vi "UHR-Fleezers Control (host) - 12.7e.vi"() -> ()   [LabVIEW 2012] (continued)
        n405 = And(x="Trap 1 ON", y=w546) -> (x .and. y?=w544:bool)
        n406 = Multiply(x=w558, y=w569) -> (x*y=w566:dbl)
        n407 = Multiply(x=w568, y=w557) -> (x*y=w564:dbl)
        n408 = Multiply(x=w567, y=w556) -> (x*y=w565:dbl)
        n409 = Multiply(x=w570, y=w555) -> (x*y=w573:dbl)
        n410 = Multiply(x=w571, y=w554) -> (x*y=w574:dbl)
        n411 = Multiply(x=w572, y=w553) -> (x*y=w575:dbl)
        n412 = call "set RF board amplitude - interlace.vi"("Board 2 Amplitude Limits"=w539, "Board 1 Amplitude Limits"=w540, "FPGA VI Reference In"=w538, "Board 2 Amplitude 3 (%)"=w575, "Board 1 Amplitude 3 (%)"=w565, "Board 2 Amplitude 2 (%)"=w574, "Board 2 Amplitude 1 (%)"=w573, "Board 1 Amplitude 2 (%)"=w564, "Board 1 Amplitude 1 (%)"=w566) -> ("error out"=w548:errorcluster, "FPGA VI Reference Out"=w549:T20)  [unwired: 1 in]
        n413 = xnode "Read/Write Control"("FPGA VI Reference In"=w549, "error in"=w548, "FB On/Off Set 1"=w544, "FB On/Off Set 2"=w541) -> ("error out"=w547:errorcluster)  [unwired: 1 out]
      }
      event "Load parameters": Value Change {
        n414 = event-data() -> ()  [unwired: 7 out]
        n415 = property on="Saved AOD Raster Scan Parameter Sets" class="Arr (strict)"() -> ("Index Values"=w586:u32[])  [unwired: 2 in, 2 out]
        n416 = Index Array(array=w586, index=0) -> (element=w583:u32)
        n417 = local write "Load parameters"(FALSE ("Load parameters")) -> ()
        n418 = Index Array(array="Saved AOD Raster Scan Parameter Sets", index=w583) -> (element=w582:T28)
        n419 = Unbundle By Name(w582) -> ("Scan Range AOD (nm) 2"=w581:dbl, "Step Size AOD (nm) 2"=w580:dbl, "Scan Speed AOD (nm/s) 2"=w579:dbl, "Number of scans (AOD) 2"=w578:u16)
        n420 = flat-sequence {
          tunnel: w581 -> [w589]
          tunnel: w580 -> [w588]
          tunnel: w579 -> [w587]
          tunnel: w578 -> [w590]
          frame #0 {
            n421 = local write "Scan Speed (nm/s)"(w587) -> ()
            n422 = local write "Scan Range (nm)"(w589) -> ()
            n423 = local write "Step Size (nm)"(w588) -> ()
          }
          frame #1 {
            n424 = property on="Number of F/B Scans (AOD)" class="DigNum (strict)"("Val(Sgnl)"=w590) -> ()  [unwired: 2 in, 2 out]
          }
        }
      }
      event "Trap 1 (ON/OFF)", "Trap 2 (ON/OFF)": Value Change {
        n425 = event-data() -> ()  [unwired: 7 out]
        n426 = property on="Trap 2 ON" class="Bool (strict)"("Val(Sgnl)"="Trap 2 (ON/OFF)") -> ()  [unwired: 2 in, 2 out]
        n427 = property on="Trap 1 ON" class="Bool (strict)"("Val(Sgnl)"="Trap 1 (ON/OFF)") -> ()  [unwired: 2 in, 2 out]
      }
      event "DIO count 1 (ticks)", "DIO count 2 (ticks)", "DIO count 3 (ticks)", "Interlace", "Number Interlace Sets", "Not-Interlacing Set", "BD 1 Delay (ticks)", "BD 2 Delay (Ticks)", "Next trap write delay (ticks)", "XY phase ext loop method", "Amp switch delay 2", "BD 2 Delay (Ticks) 2", "BD 1 Delay (ticks) 2": Value Change {
        n428 = event-data() -> ()  [unwired: 7 out]
        n429 = local read "DIO count 3 (ticks)"() -> (w611:u16)
        n430 = local read "DIO count 1 (ticks)"() -> (w613:u16)
        n431 = local read "DIO count 2 (ticks)"() -> (w612:u16)
        n432 = To Unsigned Byte Integer(number="Not-Interlacing Set") -> (unsigned 8bit integer=w602:u8)
        n433 = Add(x=w602, y=u8 1) -> (x+y=w606:u8)
        n434 = xnode "Read/Write Control"("FPGA VI Reference In"=w593, "DIO count 1 (ticks)"=w613, "DIO count 2 (ticks)"=w612, "DIO count 3 (ticks)"=w611, "Interlace ON/OFF"="Interlace", "Number Interlace Cycles"="Number Interlace Sets", "Interlace Off Parameters"=w606, "BD 1 Delay (ticks)"="BD 1 Delay (ticks)", "BD 2 Delay (Ticks)"="BD 2 Delay (Ticks)", "Next trap write delay (ticks)"="Next trap write delay (ticks)", "XY phase ext loop method"="XY phase ext loop method", "Amp switch delay 2"="Amp switch delay 2", "BD 2 Delay (Ticks) 2"="BD 2 Delay (Ticks) 2", "BD 1 Delay (ticks) 2"="BD 1 Delay (ticks) 2") -> ("error out"=w615:errorcluster)  [unwired: 1 in, 1 out]
        n435 = Build Array(w613, w612, w611) -> (w604:u16[])
        n436 = Split 1D Array(array=w604, index="Number Interlace Sets") -> (first subarray=w614:u16[])  [unwired: 1 out]
        n437 = Index Array(array=w604, index=w602) -> (element=w603:u16)
        n438 = Add Array Elements(numeric array=w614) -> (sum=w608:u16)
        n439 = Select(t=w608, s="Interlace", f=w603) -> (s? t:f=→"Total Counts (ticks)":u16)
      }
      event "Reset Feedback": Value Change {
        n440 = event-data() -> ()  [unwired: 7 out]
        n441 = Unbundle By Name("Reset Feedback") -> ("Set 1"=w619:bool, "Set 2"=w618:bool)
        n442 = xnode "Read/Write Control"("FPGA VI Reference In"=w616, "FB Reset Set 1"=w619, "FB Reset Set 2"=w618) -> ("error out"=w617:errorcluster)  [unwired: 1 in, 1 out]
      }
      event "Trap Intensity PID Gains": Value Change {
        n443 = event-data() -> ()  [unwired: 7 out]
        n444 = Unbundle By Name("Trap Intensity PID Gains") -> ("proportional gain (Kc)"=w624:i16, "integral gain (Kc*Ts/Ti)"=w623:i16, "derivative gain (Kc*Td/Ts)"=w622:i16)
        n445 = xnode "Read/Write Control"("FPGA VI Reference In"=w621, "P1"=w624, "I1"=w623, "D1"=w622) -> ("error out"=w626:errorcluster)  [unwired: 1 in, 1 out]
      }
      event "AI2 to Setpoint", "Setpoints (V)": Value Change {
        n446 = event-data() -> ()  [unwired: 7 out]
        n447 = xnode "Read/Write Control"("FPGA VI Reference In"=w627) -> ("FPGA VI Reference Out"=w630:T20, "error out"=w629:errorcluster, "AI2 Y Sum Set 1"=w637:i16, "AI2 Y Sum Set 2"=w636:i16)  [unwired: 1 in]
        n448 = Cluster To Array(cluster="AI2 to Setpoint") -> (array=w640:bool[])
        n449 = local read "AI2 (V)"() -> (w638:cluster{"Set 1":dbl, "Set 2":dbl})
        n450 = Or Array Elements(Boolean array=w640) -> (logical OR=w641:bool)
        n451 = Bundle By Name(cluster=w638, "Set 1"=w637, "Set 2"=w636) -> (w635:cluster{"Set 1":dbl, "Set 2":dbl})
        n452 = Divide(x=w635, y=3276.7) -> (x/y=w634:cluster{"Set 1":dbl, "Set 2":dbl})
        "AI2 (V)" <- w634
        n453 = case shown="True" w641 {
          tunnel: [w644 w661] -> w633
          tunnel: "AI2 to Setpoint" -> [_ w657]
          tunnel: "Setpoints (V)" -> [w645 w660]
          tunnel: w634 -> [_ w654]
          frame False {
            n454 = Multiply(x=3276.7, y=w645) -> (x*y=w646:cluster{"Set 1":dbl, "Set 2":dbl})
            n455 = To Word Integer(number=w646) -> (16bit integer=w644:cluster{"Set 1":i16, "Set 2":i16})
          }
          frame True {
            n456 = Unbundle By Name(w654) -> ("Set 1"=w653:dbl, "Set 2"=w652:dbl)
            n457 = Unbundle By Name(w660) -> ("Set 1"=w659:dbl, "Set 2"=w658:dbl)
            n458 = Unbundle By Name(w657) -> ("Set 1"=w656:bool, "Set 2"=w655:bool)
            n459 = Select(t=w653, s=w656, f=w659) -> (s? t:f=w651:dbl)
            n460 = Select(t=w652, s=w655, f=w658) -> (s? t:f=w650:dbl)
            n461 = Bundle By Name(cluster=w660, "Set 1"=w651, "Set 2"=w650) -> (w648:cluster{"Set 1":dbl, "Set 2":dbl})
            n462 = local write "Setpoints (V)"(w648) -> ()
            n463 = Multiply(x=3276.7, y=w648) -> (x*y=w649:cluster{"Set 1":dbl, "Set 2":dbl})
            n464 = To Word Integer(number=w649) -> (16bit integer=w661:cluster{"Set 1":i16, "Set 2":i16})
          }
        }
        n465 = Unbundle By Name(w633) -> ("Set 1"=w632:i16, "Set 2"=w631:i16)
        n466 = xnode "Read/Write Control"("FPGA VI Reference In"=w630, "error in"=w629, "FB Setpoint Set 1"=w632, "FB Setpoint Set 2"=w631) -> ("error out"=w628:errorcluster)  [unwired: 1 out]
      }
      event "+ phase (GI)", "- phase (GI)", "+ phase (GI) 2", "- phase (GI) 2", "+ phase (RI)", "- phase (RI)", "+ phase (Green FB)", "- phase (Green FB)": Value Change {
        n467 = event-data() -> ()  [unwired: 7 out]
        n468 = Or(x="+ phase (GI)", y="- phase (GI)") -> (x .or. y?=w697:bool)
        n469 = Negate(x="Phase adj. (GI)") -> (-x=w702:i16)
        n470 = Select(t=w702, s="+ phase (GI)", f="Phase adj. (GI)") -> (s? t:f=w701:i16)
        n471 = Or(x="+ phase (GI) 2", y="- phase (GI) 2") -> (x .or. y?=w688:bool)
        n472 = Negate(x="Phase adj. (GI) 2") -> (-x=w693:i16)
        n473 = Select(t=w693, s="+ phase (GI) 2", f="Phase adj. (GI) 2") -> (s? t:f=w689:i16)
        n474 = Negate(x="Phase adj. (RI)") -> (-x=w687:i16)
        n475 = Or(x="+ phase (RI)", y="- phase (RI)") -> (x .or. y?=w683:bool)
        n476 = Select(t=w687, s="+ phase (RI)", f="Phase adj. (RI)") -> (s? t:f=w682:i16)
        n477 = Or(x="+ phase (Green FB)", y="- phase (Green FB)") -> (x .or. y?=w676:bool)
        n478 = Negate(x="Phase adj. (Green FB)") -> (-x=w681:i16)
        n479 = Select(t=w681, s="+ phase (Green FB)", f="Phase adj. (Green FB)") -> (s? t:f=w677:i16)
        n480 = Negate(x="Phase adj. (BI AO)") -> (-x=w675:i16)
        n481 = Or(x="+ phase (BI AO)", y="- phase (BI AO)") -> (x .or. y?=w665:bool)
        n482 = Select(t=w675, s="+ phase (BI AO)", f="Phase adj. (BI AO)") -> (s? t:f=w667:i16)
        n483 = Negate(x="Phase adj. (BI DO)") -> (-x=w671:i16)
        n484 = Or(x="+ phase (BI DO)", y="- phase (BI DO)") -> (x .or. y?=w664:bool)
        n485 = Select(t=w671, s="+ phase (BI DO)", f="Phase adj. (BI DO)") -> (s? t:f=w666:i16)
        n486 = xnode "Read/Write Control"("FPGA VI Reference In"=w663, "Phase count adjustment (GI)"=w701, "Phase count adjustment (GI) 2"=w689, "Phase count adjustment (RI)"=w682, "Phase count adjustment (Green FB)"=w677, "Phase count adjustment (BI AO)"=w667, "Phase count adjustment (BI D)"=w666) -> ("FPGA VI Reference Out"=w699:T20, "error out"=w700:errorcluster)  [unwired: 1 in]
        n487 = xnode "Read/Write Control"("FPGA VI Reference In"=w699, "error in"=w700, "+ phase (GI)"=w697, "+ phase (GI) 2"=w688, "+ phase (RI)"=w683, "+ phase (Green FB)"=w676, "+ phase (BI AO)"=w665, "+ phase (BI D)"=w664) -> ("error out"=w698:errorcluster)  [unwired: 1 out]
      }
      event "Green Laser ON/OFF", "Red Laser ON/OFF", "Blue Laser ON/OFF": Value Change {
        # "This loop shouldn't be initialized.  The main 'laser ON' settings should dominate and set the others."
        n488 = event-data() -> ()  [unwired: 7 out]
        n489 = property on="Red Laser ON" class="Bool (strict)"("Val(Sgnl)"="Red Laser ON/OFF") -> ()  [unwired: 2 in, 2 out]
        n490 = property on="Blue Laser ON" class="Bool (strict)"("Val(Sgnl)"="Blue Laser ON/OFF") -> ()  [unwired: 2 in, 2 out]
        n491 = property on="Green Laser ON" class="Bool (strict)"("Val(Sgnl)"="Green Laser ON/OFF") -> ()  [unwired: 2 in, 2 out]
      }
      event "Laser interlacing mode", "Green Laser ON", "Red Laser ON", "Blue Laser ON": Value Change {
        n492 = event-data() -> ()  [unwired: 7 out]
        n493 = local write "Green Laser ON/OFF"("Green Laser ON") -> ()
        n494 = local write "Blue Laser ON/OFF"("Blue Laser ON") -> ()
        n495 = local write "Red Laser ON/OFF"("Red Laser ON") -> ()
        n496 = case shown="True" "Green Laser ON" {
          tunnel: "Laser interlacing mode" -> [_ w738]
          tunnel: [enum32{"Laser ON", "Laser OFF", "Interlace"}."Laser OFF" ("Green laser mode") w738] -> w716
          tunnel: [FALSE w734] -> w715
          frame False {
          }
          frame True {
            n497 = local read "Green FB On/Off"() -> (w735:bool)
            n498 = Equal?(x=w738, y=enum32{"Laser ON", "Laser OFF", "Interlace"}."Interlace") -> (x = y?=w736:bool)
            n499 = And(x=w736, y=w735) -> (x .and. y?=w734:bool)
          }
        }
        n500 = case shown="True" "Red Laser ON" {
          tunnel: "Laser interlacing mode" -> [_ w731]
          tunnel: [enum32{"Laser ON", "Laser OFF", "Interlace"}."Laser OFF" ("Green laser mode") w731] -> w712
          tunnel: [FALSE w727] -> w711
          frame False {
          }
          frame True {
            n501 = local read "Red FB On/Off"() -> (w728:bool)
            n502 = Equal?(x=w731, y=enum32{"Laser ON", "Laser OFF", "Interlace"}."Interlace") -> (x = y?=w729:bool)
            n503 = And(x=w729, y=w728) -> (x .and. y?=w727:bool)
          }
        }
        n504 = case shown="True" "Blue Laser ON" {
          tunnel: "Laser interlacing mode" -> [_ w722]
          tunnel: [enum32{"Laser ON", "Laser OFF", "Interlace"}."Laser OFF" ("Green laser mode") w722] -> w708
          tunnel: [FALSE w720] -> w707
          frame False {
          }
          frame True {
            n505 = local read "Blue FB On/Off"() -> (w721:bool)
            n506 = Equal?(x=w722, y=enum32{"Laser ON", "Laser OFF", "Interlace"}."Interlace") -> (x = y?=w723:bool)
            n507 = And(x=w723, y=w721) -> (x .and. y?=w720:bool)
          }
        }
        n508 = xnode "Read/Write Control"("FPGA VI Reference In"=w706, "Operating Mode"=w716, "Operating Mode 2"=w716, "Green FB On/Off"=w715, "Red Laser Operating Mode"=w712, "RI Operating Mode 2"=w712, "Red FB On/Off"=w711, "BI Operating Mode (AO)"=w708, "Blue Laser Operating Mode (D)"=w708, "Blue FB On/Off"=w707) -> ("error out"=w717:errorcluster)  [unwired: 1 in, 1 out]
      }
      event "Invert laser interlacing": Value Change {
        n509 = event-data() -> ()  [unwired: 7 out]
        n510 = xnode "Read/Write Control"("FPGA VI Reference In"=w739, "Invert GI"="Invert laser interlacing", "Invert GI 2"="Invert laser interlacing", "Invert RI"="Invert laser interlacing", "Invert RI 2"="Invert laser interlacing", "Invert BI (AO)"="Invert laser interlacing", "Invert BI (D)"="Invert laser interlacing") -> ("error out"=w741:errorcluster)  [unwired: 1 in, 1 out]
      }
      event "Green FB Setpoint (mV)", "Green FB Gains", "Green FB On/Off", "Green Intensity % (FB OFF)", "Green int current ON count adj": Value Change {
        n511 = event-data() -> ()  [unwired: 7 out]
        n512 = local read "Green FB Setpoint (mV)"() -> (w753:dbl)
        n513 = Multiply(x=w753, y=3.2767) -> (x*y=w752:dbl)
        n514 = local read "Green Intensity % (FB OFF)"() -> (w756:dbl)
        n515 = Multiply(x=w756, y=655.35) -> (x*y=w757:dbl)
        n516 = To Unsigned Word Integer(number=w757) -> (unsigned 16bit integer=w755:u16)
        n517 = local read "Green int current ON count adj"() -> (w759:u32)
        n518 = local read "Laser interlacing mode"() -> (w749:enum32{"Laser ON", "Laser OFF", "Interlace"})
        n519 = local read "Green FB Gains"() -> (w746:T9)
        n520 = local read "Green Laser ON"() -> (w750:bool)
        n521 = local read "Green FB On/Off"() -> (w760:bool)
        n522 = Equal?(x=w749, y=enum32{"Laser ON", "Laser OFF", "Interlace"}."Interlace") -> (x = y?=w747:bool)
        n523 = Unbundle By Name(w746) -> ("proportional gain (Kc)"=w745:i16, "integral gain (Kc*Ts/Ti)"=w744:i16, "derivative gain (Kc*Td/Ts)"=w743:i16)
        n524 = Compound Arithmetic op=AND(w747, w760, w750) -> (w751:bool)
        n525 = xnode "Read/Write Control"("FPGA VI Reference In"=w742, "Green FB Setpoint"=w752, "Green FB On/Off"=w751, "Current Out"=w755, "Green int current ON count adj"=w759, "P3"=w745, "I3"=w744, "D3"=w743) -> ("error out"=w761:errorcluster)  [unwired: 1 in, 1 out]
      }
      event "Blue FB Setpoint (mV)", "Blue FB Gains", "Blue FB On/Off", "Blue Intensity % (FB OFF)", "Blue int AO ON count adjust": Value Change {
        # "16 bit analog out"
        n526 = event-data() -> ()  [unwired: 7 out]
        n527 = Multiply(x="Blue FB Setpoint (mV)", y=3.2767) -> (x*y=w776:dbl)
        n528 = Multiply(x="Blue Intensity % (FB OFF)", y=655.35) -> (x*y=w779:dbl)
        n529 = To Unsigned Word Integer(number=w779) -> (unsigned 16bit integer=w778:u16)
        n530 = local read "Laser interlacing mode"() -> (w774:enum32{"Laser ON", "Laser OFF", "Interlace"})
        n531 = Unbundle By Name("Blue FB Gains") -> ("proportional gain (Kc)"=w771:i16, "integral gain (Kc*Ts/Ti)"=w770:i16, "derivative gain (Kc*Td/Ts)"=w769:i16)
        n532 = local read "Blue Laser ON"() -> (w763:bool)
        n533 = Equal?(x=w774, y=enum32{"Laser ON", "Laser OFF", "Interlace"}."Interlace") -> (x = y?=w772:bool)
        n534 = Compound Arithmetic op=AND(w772, "Blue FB On/Off", w763) -> (w775:bool)
        n535 = xnode "Read/Write Control"("FPGA VI Reference In"=w762, "Blue FB Setpoint"=w776, "Blue FB On/Off"=w775, "BI Current Out"=w778, "Blue current ON count adj (AO)"="Blue int AO ON count adjust", "P5"=w771, "I5"=w770, "D5"=w769) -> ("error out"=w781:errorcluster)  [unwired: 1 in, 1 out]
      }
      event "Red FB Setpoint (mV)", "Red FB Gains", "Red FB On/Off", "Red Intensity % (FB OFF)": Value Change {
        n536 = event-data() -> ()  [unwired: 7 out]
        n537 = local read "Red FB Setpoint (mV)"() -> (w794:dbl)
        n538 = Multiply(x=w794, y=3.2767) -> (x*y=w793:dbl)
        n539 = local read "Red Intensity % (FB OFF)"() -> (w783:dbl)
        n540 = Multiply(x=w783, y=655.35) -> (x*y=w797:dbl)
        n541 = To Unsigned Word Integer(number=w797) -> (unsigned 16bit integer=w796:u16)
        n542 = local read "Laser interlacing mode"() -> (w790:enum32{"Laser ON", "Laser OFF", "Interlace"})
        n543 = local read "Red FB Gains"() -> (w787:T9)
        n544 = local read "Red Laser ON"() -> (w791:bool)
        n545 = local read "Red FB On/Off"() -> (w799:bool)
        n546 = Equal?(x=w790, y=enum32{"Laser ON", "Laser OFF", "Interlace"}."Interlace") -> (x = y?=w788:bool)
        n547 = Unbundle By Name(w787) -> ("proportional gain (Kc)"=w786:i16, "integral gain (Kc*Ts/Ti)"=w785:i16, "derivative gain (Kc*Td/Ts)"=w784:i16)
        n548 = Compound Arithmetic op=AND(w788, w799, w791) -> (w792:bool)
        n549 = xnode "Read/Write Control"("FPGA VI Reference In"=w782, "Red FB Setpoint"=w793, "Red FB On/Off"=w792, "RI Current Out"=w796, "P4"=w786, "I4"=w785, "D4"=w784) -> ("error out"=w800:errorcluster)  [unwired: 1 in, 1 out]
      }
      event "+ phase (APD 1 Gate)", "- phase (APD 1 Gate)", "+ phase (APD 2 Gate)", "- phase (APD 2 Gate)", "+ phase (APD 3 Gate)", "- phase (APD 3 Gate)", "+ phase (APD Acq)", "- phase (APD Acq)": Value Change {
        n550 = event-data() -> ()  [unwired: 7 out]
        n551 = local read "Phase Adj. (APD 1 Gate)"() -> (w821:i16)
        n552 = Or(x="- phase (APD 1 Gate)", y="+ phase (APD 1 Gate)") -> (x .or. y?=w823:bool)
        n553 = Negate(x=w821) -> (-x=w828:i16)
        n554 = Select(t=w828, s="+ phase (APD 1 Gate)", f=w821) -> (s? t:f=w827:i16)
        n555 = local read "Phase Adj. (APD 2 Gate)"() -> (w818:i16)
        n556 = Or(x="- phase (APD 2 Gate)", y="+ phase (APD 2 Gate)") -> (x .or. y?=w816:bool)
        n557 = Negate(x=w818) -> (-x=w820:i16)
        n558 = Select(t=w820, s="+ phase (APD 2 Gate)", f=w818) -> (s? t:f=w817:i16)
        n559 = Negate(x="Phase Adj. (APD 3 Gate)") -> (-x=w815:i16)
        n560 = Or(x="- phase (APD 3 Gate)", y="+ phase (APD 3 Gate)") -> (x .or. y?=w811:bool)
        n561 = Select(t=w815, s="+ phase (APD 3 Gate)", f="Phase Adj. (APD 3 Gate)") -> (s? t:f=w812:i16)
        n562 = local read "Phase Adj. (APD Acq)"() -> (w809:i16)
        n563 = Or(x="- phase (APD Acq)", y="+ phase (APD Acq)") -> (x .or. y?=w807:bool)
        n564 = Negate(x=w809) -> (-x=w810:i16)
        n565 = Select(t=w810, s="+ phase (APD Acq)", f=w809) -> (s? t:f=w808:i16)
        n566 = xnode "Read/Write Control"("FPGA VI Reference In"=w801, "Phase count adjustment (APD 1 Gate)"=w827, "Phase count adjustment (APD 2 Gate)"=w817, "Phase count adjustment (APD 3 Gate)"=w812, "Phase Count Adjustment (APD Acq)"=w808) -> ("FPGA VI Reference Out"=w825:T20, "error out"=w826:errorcluster)  [unwired: 1 in]
        n567 = xnode "Read/Write Control"("FPGA VI Reference In"=w825, "error in"=w826, "+ phase (APD 1 Gate)"=w823, "+ phase (APD 2 Gate)"=w816, "+ phase (APD 3 Gate)"=w811, "+ phase (APD Acq)"=w807) -> ("error out"=w824:errorcluster)  [unwired: 1 out]
      }
      event "Invert APD Gate", "APD Gate ON Count", "APD Gate OFF Count", "APD Gate", "APD Integration Time (s)", "APD AO Scale Factor", "Duty Frequency (ON 1/N cycles)", "Interlace ON count", "Interlace OFF count": Value Change {
        n568 = event-data() -> ()  [unwired: 7 out]
        n569 = Add(x="Interlace ON count", y="Interlace OFF count") -> (x+y=w835:u16)
        n570 = Add(x="APD Gate ON Count", y="APD Gate OFF Count") -> (x+y=w846:u16)
        n571 = Multiply(x="Duty Frequency (ON 1/N cycles)", y=w835) -> (x*y=w831:u16)
        "Green AI Count" <- w831
        "Red AI Count" <- w831
        "Blue AI Count" <- w831
        n572 = Subtract(x=w831, y="Interlace ON count") -> (x-y=w834:u16)
        n573 = Multiply(x=w846, y="Duty Frequency (ON 1/N cycles)") -> (x*y=w845:u16)
        n574 = Subtract(x=w845, y="APD Gate ON Count") -> (x-y=w844:u16)
        n575 = local read "DMA Update Period (s)"() -> (w847:dbl)
        n576 = Multiply(x="APD Integration Time (s)", y=40000000.0) -> (x*y=w851:dbl)
        n577 = Reciprocal(x="APD Integration Time (s)") -> (1/x=→"APD Acq Rate (Hz)":dbl)
        n578 = To Unsigned Long Integer(number=w851) -> (unsigned 32bit integer=w837:u32)
        "APD Int. Count" <- w837
        n579 = local read "Number of APDs"() -> (w830:u8)
        n580 = Divide(x=w847, y="APD Integration Time (s)") -> (x/y=w849:dbl)
        n581 = Multiply(x=w830, y=w849) -> (x*y=w848:dbl)
        n582 = local write "APD Samples/FIFO Acq."(w849) -> ()
        n583 = local write "APD Elements/DMA read"(w848) -> ()
        n584 = xnode "Read/Write Control"("FPGA VI Reference In"=w829, "Invert APD Gate"="Invert APD Gate", "APD Gate ON Count"="APD Gate ON Count", "APD Gate OFF Count"=w844, "APD Acq Rate Count"=w837, "APD Gate Operating Mode"="APD Gate", "APD AO scale factor"="APD AO Scale Factor", "Green interlace ON count"="Interlace ON count", "Green interlace OFF count"=w834, "Green interlace ON count 2"="Interlace ON count", "Green interlace OFF count 2"=w834, "Green FB Count"=w831, "Red interlace ON count"="Interlace ON count", "Red interlace OFF count"="Interlace OFF count", "Blue ON count (AO)"="Interlace ON count", "Blue OFF count (AO)"="Interlace OFF count", "Blue interlace OFF count (D)"="Interlace OFF count", "Blue interlace ON count (D)"="Interlace ON count") -> ("error out"=w853:errorcluster)  [unwired: 1 in, 1 out]
      }
      event "Neg. TTrig FPGA": Value Change {
        n585 = event-data() -> ()  [unwired: 7 out]
        n586 = xnode "Read/Write Control"("FPGA VI Reference In"=w854, "TTrig Negate Pos"="Neg. TTrig FPGA") -> ()  [unwired: 1 in, 2 out]
      }
      event "Test ttrig": Value Change {
        n587 = event-data() -> ()  [unwired: 7 out]
        n588 = xnode "Read/Write Control"("FPGA VI Reference In"=w856, "TTrig?"=TRUE) -> ("error out"=w858:errorcluster)  [unwired: 1 in, 1 out]
      }
      event "Number of F/B Scans (AOD)", "Scan Speed (nm/s)", "Scan BD", "Initial delta (MHz)", "Step Size (nm)", "Scan Range (nm)": Value Change {
        w922 = 123.0  # AOM cal (nm/MHz)
        n589 = event-data() -> ()  [unwired: 7 out]
        n590 = local read "BD 1 Frequency 1 (MHz)"() -> (w905:dbl)
        n591 = local read "AOM X Cal (nm/MHz)"() -> (w897:dbl)
        n592 = local read "X RF Frequency Limits (MHz)"() -> (w909:T16)
        n593 = local read "Y RF Frequency Limits (MHz)"() -> (w906:T16)
        n594 = local read "BD 2 Frequency 1 (MHz)"() -> (w911:dbl)
        n595 = Negate(x="Scan Range (nm)") -> (-x=w875:dbl)
        n596 = Divide(x=w875, y=w897) -> (x/y=w879:dbl)
        n597 = Select(t=w909, s="Scan BD", f=w906) -> (s? t:f=w908:T16)
        n598 = Select(t=w905, s="Scan BD", f=w911) -> (s? t:f=w910:dbl)
        n599 = Unbundle By Name(w908) -> ("Maximum"=w917:dbl, "Minimum"=w916:dbl)
        n600 = Add(x=w879, y=w910) -> (x+y=w914:dbl)
        n601 = Divide(x=w875, y="Step Size (nm)") -> (x/y=w894:dbl)
        n602 = Divide(x="Step Size (nm)", y=w897) -> (x/y=w903:dbl)
        n603 = Absolute Value(x=w894) -> (abs(x)=w878:dbl)
        n604 = Sign(1:w875) -> (0:w876:dbl)
        n605 = In Range and Coerce(upper limit=w917, x=w914, lower limit=w916) -> (coerced(x)=w913:dbl, In Range?=w915:bool)
        n606 = To Unsigned Quad Integer(1:w878) -> (0:w893:u64)
        "Scan steps (AOD)" <- w893
        n607 = call "IR AOM freq to word.vi"("Frequency In (MHz)"=w903) -> ("Frequency Word Out (double)"=w900:dbl)
        n608 = Multiply(x=w876, y=w900) -> (x*y=w877:dbl)
        n609 = Subtract(x=w914, y=w913) -> (x-y=w912:dbl)
        n610 = To Quad Integer(1:w877) -> (0:w899:i64)
        "Incr. int (AOD)" <- w899
        n611 = Subtract(x=w879, y=w912) -> (x-y=w898:dbl)
        "Scan Range (MHz)" <- w898
        n612 = Select(t=w879, s=w915, f=w898) -> (s? t:f=w918:dbl)
        n613 = Multiply(x=w898, y=w897) -> (x*y=w896:dbl)
        n614 = Decrement(x=w893) -> (x-1=w946:u64)
        n615 = Negate(x=w896) -> (-x=w892:dbl)
        n616 = local write "Scan Range (nm)"(w892) -> ()
        n617 = Divide(x=w918, y=w946) -> (x/y=w902:dbl)
        "Scan Increment (MHz)" <- w902
        n618 = call "IR AOM freq to word.vi"("Frequency In (MHz)"=w902) -> ("Frequency Word Out (double)"=w901:dbl)
        n619 = Divide(x="Step Size (nm)", y="Scan Speed (nm/s)") -> (x/y=w889:dbl)
        n620 = To Quad Integer(1:w901) -> ()  [unwired: 1 out]
        n621 = local read "Number Interlace Sets"() -> (w873:u8)
        n622 = local read "AI Count (ticks)"() -> (w874:u16)
        n623 = local read "Total Counts (ticks)"() -> (w872:u16)
        n624 = local read "# Samples/trap"() -> (w904:u32)
        n625 = Multiply(x=w874, y=w873) -> (x*y=w871:u16)
        n626 = Divide(x=w872, y=w871) -> (x/y=w870:dbl)
        n627 = Select(t=w905, s="Scan BD", f=w911) -> (s? t:f=w943:dbl)
        "Initial freq. (MHz)" <- w943
        n628 = Add(x=w918, y=w943) -> (x+y=→"Final freq. (MHz)":dbl)
        n629 = Divide(x=w872, y=40000000.0) -> (x/y=w888:dbl)
        n630 = Divide(x=w889, y=w888) -> (x/y=w887:dbl)
        n631 = To Unsigned Quad Integer(1:w887) -> (0:w862:u64)
        n632 = Quotient & Remainder(x=w862, y=u64 2) -> (x-y*floor(x/y)=w866:u64)  [unwired: 1 out]
        n633 = Equal?(x=w866, y=u64 0) -> (x = y?=w864:bool)
        n634 = Decrement(x=w862) -> (x-1=w863:u64)
        n635 = Select(t=w862, s=w864, f=w863) -> (s? t:f=w861:u64)
        "Cycles/step (AOD)" <- w861
        n636 = xnode "Read/Write Control"("FPGA VI Reference In"=w860, "Scan steps"=w893, "Number of scans"="Number of F/B Scans (AOD)", "Cycles per step"=w861, "Scan freq.  increment"=w899, "Scan BD"="Scan BD") -> ("error out"=w952:errorcluster)  [unwired: 1 in, 1 out]
        n637 = Multiply(x=w893, y=w861) -> (x*y=w947:u64)
        n638 = Multiply(x=w947, y=u64 2) -> (x*y=w869:u64)
        n639 = Multiply(x=w870, y=w869) -> (x*y=w868:dbl)
        "Data points/scan (f/b)" <- w868
        n640 = Multiply(x=w868, y="Number of F/B Scans (AOD)") -> (x*y=w950:dbl)
        "Data points/scans" <- w950
        n641 = Divide(x=w950, y=w904) -> (x/y=→"N sets should be saved":dbl)
        n642 = Multiply(x=w947, y=w888) -> (x*y=w886:dbl)
        "Time/Scan (s) (AOD)" <- w886
        n643 = Select(t=w918, s="Scan BD", f=0.0) -> (s? t:f=w944:dbl)
        n644 = Select(t=0.0, s="Scan BD", f=w918) -> (s? t:f=w940:dbl)
        n645 = local read "BD 2 Frequency 2 (MHz)"() -> (w936:dbl)
        n646 = local read "BD 1 Frequency 2 (MHz)"() -> (w939:dbl)
        n647 = Add(x=w940, y=w911) -> (x+y=w937:dbl)
        n648 = Add(x=w905, y=w944) -> (x+y=w938:dbl)
        n649 = Multiply(x=w886, y=2.0) -> (x*y=w885:dbl)
        n650 = Multiply(x=w885, y="Number of F/B Scans (AOD)") -> (x*y=w882:dbl)
        n651 = Divide(x=w882, y=60.0) -> (x/y=→"Time to Finish All (min)":dbl)
        n652 = Add(x="Trap 2 Bead Size (nm)", y="Trap 1 Bead Size (nm)") -> (x+y=w926:dbl)
        n653 = Divide(x=w926, y=2.0) -> (x/y=w920:dbl)
        n654 = local read "Initial delta (MHz)"() -> (w923:dbl)
        n655 = Subtract(x=w937, y=w936) -> (x-y=w934:dbl)
        n656 = Subtract(x=w938, y=w939) -> (x-y=w935:dbl)
        n657 = Square(x=w934) -> (x^2=w933:dbl)
        n658 = Square(x=w935) -> (x^2=w932:dbl)
        n659 = Add(x=w932, y=w933) -> (x+y=w931:dbl)
        n660 = Square Root(x=w931) -> (sqrt(x)=w930:dbl)
        "Final delta (MHz)" <- w930
        n661 = Multiply(x=w922, y=w930) -> (x*y=w929:dbl)
        n662 = Multiply(x=w923, y=w922) -> (x*y=w921:dbl)
        n663 = Subtract(x=w921, y=w920) -> (x-y=→"Initial sep (nm)":dbl)
        n664 = Subtract(x=w929, y=w920) -> (x-y=→"Final sep (nm)":dbl)
      }
      event "Freq or Amp switch first", "Swap F1 and F2", "Freq switch delay", "Amp switch delay": Value Change {
        n665 = event-data() -> ()  [unwired: 7 out]
        n666 = local read "Amp switch delay"() -> (w954:u16)
        n667 = local read "Swap F1 and F2"() -> (w955:bool)
        n668 = xnode "Read/Write Control"("FPGA VI Reference In"=w953, "Swap F1 and F2"=w955, "Amp switch delay"=w954) -> ("error out"=w956:errorcluster)  [unwired: 1 in, 1 out]
      }
      event "Scan steps (MCL)", "Number of scans (MCL)", "Scan Range (V)\n(of steps)", "2D or 1D Scan", "N APD Samp/step", "Fast Scan Dir", "Continuous MCL Scanning", "Scan lines (y)": Value Change {
        w959 = 32767.0 ("y")
        n669 = event-data() -> ()  [unwired: 7 out]
        n670 = Select(t="Scan lines (y)", s="2D or 1D Scan", f="Number of scans (MCL)") -> (s? t:f=w964:u64)
        n671 = Decrement(x="Scan steps (MCL)") -> (x-1=w980:u64)
        n672 = Divide(x="Scan Range (V)\n(of steps)", y=w980) -> (x/y=w979:dbl)
        "Desired Scan Incr (V)" <- w979
        n673 = local read "APD Integration Time (s)"() -> (w972:dbl)
        n674 = Multiply(x=w979, y=w959) -> (x*y=w988:dbl)
        n675 = Divide(x=w988, y=10.0) -> (x/y=w978:dbl)
        "Desired incr (int)" <- w978
        n676 = local read "Update Count (MCL)"() -> (w984:u32)
        n677 = Round Toward -Infinity(1:w978) -> (0:w987:dbl)
        n678 = To Word Integer(number=w987) -> (16bit integer=w962:i16)
        "Actual Incr. int (MCL)" <- w962
        n679 = Multiply(x=w972, y=40000000.0) -> (x*y=w985:dbl)
        n680 = Divide(x=w985, y=w984) -> (x/y=w983:dbl)
        n681 = Multiply(x=i16 10, y=w962) -> (x*y=w960:i16)
        n682 = Multiply(x="N APD Samp/step", y=w983) -> (x*y=w982:dbl)
        "Cycles/step (MCL)" <- w982
        n683 = Divide(x=w960, y=w959) -> (x/y=→"Actual MCL Inc (V)":dbl)
        n684 = Multiply(x="N APD Samp/step", y="Scan steps (MCL)") -> (x*y=w974:dbl)
        n685 = local read "APD Samples/FIFO Acq."() -> (w971:dbl)
        n686 = Multiply(x=w974, y=u64 2) -> (x*y=w973:dbl)
        "Data points/scan (f+b)" <- w973
        n687 = Multiply(x=w973, y=w964) -> (x*y=w991:dbl)
        "Data points/scans (MCL)" <- w991
        n688 = Multiply(x=w972, y=w973) -> (x*y=w965:dbl)
        "Time/f+b scan (s) (MCL)" <- w965
        n689 = Divide(x=w991, y=w971) -> (x/y=→"N sets should be saved (MCL)":dbl)
        n690 = Multiply(x=w965, y=w964) -> (x*y=→"Total Time (s)":dbl)
        n691 = Not(x="Fast Scan Dir") -> (.not. x?=w969:bool)
        n692 = xnode "Read/Write Control"("FPGA VI Reference In"=w957, "Scan steps (MCL)"="Scan steps (MCL)", "Number of scans (MCL)"=w964, "Cycles per step (MCL)"=w982, "Scan freq.  increment (MCL)"=w962, "1D or 2D Scan?"="2D or 1D Scan", "MCL Scan Axis"=w969, "Cont. Scan (MCL)"="Continuous MCL Scanning") -> ("error out"=w993:errorcluster)  [unwired: 1 in, 1 out]
      }
      event "Read Cal": Value Change {
        w995 = 1000.0 ("y")
        n693 = event-data() -> ()  [unwired: 7 out]
        n694 = local read "Save file name"() -> (w1020:path)
        n695 = local write "Read Cal"(FALSE ("Read Cal")) -> ()
        n696 = Strip Path(path=w1020) -> (stripped path=w1019:path)  [unwired: 1 out]
        n697 = Path To String(path=w1019) -> (string=w1018:string)
        n698 = Concatenate Strings(w1018, "\\current.cal" ("string")) -> (w1016:string)
        n699 = String To Path(string=w1016) -> (path=w1015:path)
        n700 = Open/Create/Replace File(file path (use dialog)=w1015, operation (0:open)=T27."open", access (0:read/write)=enum16{"read/write", "read-only", "write-only"}."read-only") -> (refnum out=w1023:refnum<file>, error out=w1009:errorcluster)  [unwired: 1 in, 3 out]
        n701 = Deny Access(4:w1009, 7:w1023) -> (0:w1008:errorcluster, 3:w1014:refnum<file>)  [unwired: 1 out]
        n702 = Read from Binary File(5:0.0, 8:w1008, 9:T26."big-endian, network order" ("byte order (0:big-endian, network order)"), 10:-1 ("count (1)"), 11:w1014) -> (0:w1007:errorcluster, 2:w1005:dbl[], 3:w1010:refnum<file>)  [unwired: 2 out]
        n703 = Array To Cluster(array=w1005) -> (cluster=w1004:T29)
        n704 = Unbundle(w1004) -> ("[0]"=w1003:dbl, "[1]"=w1002:dbl, "[2]"=w1001:dbl, "[3]"=w1000:dbl, "[4]"=w999:dbl, "[5]"=w998:dbl)
        n705 = Close File(refnum=w1010, error in=w1007) -> (error out=→"Read cal error":errorcluster)  [unwired: 1 out]
        n706 = Multiply(x=w998, y=w995) -> (x*y=w996:dbl)
        n707 = local write "T2 kappa_x (pN/nm)"(w1000) -> ()
        n708 = local write "T1 kappa_x (pN/nm)"(w1001) -> ()
        n709 = local write "T1 alpha_x (nm/V)"(w1003) -> ()
        n710 = local write "T2 alpha_x (nm/V)"(w1002) -> ()
        n711 = Multiply(x=w999, y=w995) -> (x*y=w997:dbl)
        n712 = local write "T1 offset_x (mV)"(w997) -> ()
        n713 = local write "T2 offset_x (mV)"(w996) -> ()
      }
      event "Abort MCL Scan": Value Change {
        n714 = event-data() -> ()  [unwired: 7 out]
        n715 = local write "MCL Scanning"(FALSE ("MCL Scanning")) -> ()
        n716 = xnode "Read/Write Control"("FPGA VI Reference In"=w1024, "Abort scan (MCL)"="Abort MCL Scan") -> ("error out"=w1027:errorcluster)  [unwired: 1 in, 1 out]
      }
      event "Update Count (MCL)": Value Change {
        n717 = event-data() -> ()  [unwired: 7 out]
        n718 = xnode "Read/Write Control"("FPGA VI Reference In"=w1028, "MCL count"="Update Count (MCL)") -> ("error out"=w1030:errorcluster)  [unwired: 1 in, 1 out]
      }
      event "+ phase (MCL)", "- phase (MCL)": Value Change {
        n719 = event-data() -> ()  [unwired: 7 out]
        n720 = Or(x="- phase (MCL)", y="+ phase (MCL)") -> (x .or. y?=w1034:bool)
        n721 = Negate(x="Phase adjust (MCL)") -> (-x=w1040:i16)
        n722 = Select(t=w1040, s="+ phase (MCL)", f="Phase adjust (MCL)") -> (s? t:f=w1038:i16)
        n723 = xnode "Read/Write Control"("FPGA VI Reference In"=w1031, "Phase count adjustment (MCL)"=w1038) -> ("FPGA VI Reference Out"=w1035:T20, "error out"=w1036:errorcluster)  [unwired: 1 in]
        n724 = xnode "Read/Write Control"("FPGA VI Reference In"=w1035, "error in"=w1036, "+ phase (MCL)"=w1034) -> ("error out"=w1033:errorcluster)  [unwired: 1 out]
      }
      event "Abort AOD Scan": Value Change {
        n725 = event-data() -> ()  [unwired: 7 out]
        n726 = xnode "Read/Write Control"("FPGA VI Reference In"=w1041, "Abort scan"="Abort AOD Scan") -> ("error out"=w1043:errorcluster)  [unwired: 1 in, 1 out]
      }
      event "Continuous AOD Scanning": Value Change {
        n727 = event-data() -> ()  [unwired: 7 out]
        n728 = xnode "Read/Write Control"("FPGA VI Reference In"=w1044, "Cont. Scan"="Continuous AOD Scanning") -> ("error out"=w1046:errorcluster)  [unwired: 1 in, 1 out]
      }
      event "Index": Value Change {
        n729 = event-data() -> ()  [unwired: 7 out]
        n730 = call "Create new save file.vi"("Insert"="", "Ext"=".dat" ("string"), "Index In"="Index") -> ("Path Out"=→"Save file name":path, "Index Out"=w1047:dbl)
        "Save index" <- w1047
        n731 = local write "Index"(w1047) -> ()
      }
      event "AO1", "AO2": Value Change {
        w1061 = 10.0 ("y")
        w1060 = 32767.0 ("y")
        n732 = event-data() -> ()  [unwired: 7 out]
        n733 = local read "AO2"() -> (w1059:dbl)
        n734 = local read "AO1"() -> (w1056:dbl)
        n735 = Multiply(x=w1056, y=w1060) -> (x*y=w1055:dbl)
        n736 = Multiply(x=w1059, y=w1060) -> (x*y=w1058:dbl)
        n737 = Divide(x=w1055, y=w1061) -> (x/y=w1054:dbl)
        n738 = Divide(x=w1058, y=w1061) -> (x/y=w1057:dbl)
        n739 = To Word Integer(number=w1054) -> (16bit integer=w1062:i16)
        n740 = To Word Integer(number=w1057) -> (16bit integer=w1063:i16)
        n741 = xnode "Read/Write Control"("FPGA VI Reference In"=w1052, "AO1"=w1062, "AO2"=w1063) -> ("error out"=w1053:errorcluster)  [unwired: 1 in, 1 out]
      }
      event "Inject Pump 1": Value Change {
        n742 = event-data() -> ()  [unwired: 7 out]
        n743 = local read "Use Harvard pumps\nfor beads (else Chemyx)"() -> (w1065:bool)
        n744 = case shown="True" w1065 {
          tunnel: "Inject Pump 1" -> [w1069 w1107]
          tunnel: w1064 -> [_ w1108]
          frame False {
            n745 = local read "Pump write delay (ms)"() -> (w1068:dbl)
            n746 = local read "Chemyx Syringe Pump Serial Port"() -> (w1067:refnum<visa-resource-name>)
            n747 = case shown="True" w1069 {
              tunnel: w1068 -> [w1075 w1089]
              tunnel: w1067 -> [w1072 w1088]
              frame False {
                n748 = flat-sequence {
                  tunnel: w1072 -> [w1076]
                  tunnel: [w1076] -> w1073
                  tunnel: w1075 -> [_]
                  tunnel: [w1079] -> w1074
                  tunnel: w1073 -> [w1079]
                  tunnel: w1074 -> [w1080]
                  tunnel: [w1080] -> w1070
                  tunnel: [w1082] -> w1071
                  tunnel: w1070 -> [w1082]
                  tunnel: w1071 -> [w1084]
                  frame #0 {
                    n749 = call "Write to pump.vi"("string"="enter pump1", "VISA resource name"=w1076) -> ()  [unwired: 1 out]
                  }
                  frame #1 {
                    n750 = Wait (ms)(milliseconds to wait="Pump pause delay (ms)") -> ()  [unwired: 1 out]
                  }
                  frame #2 {
                    n751 = call "Write to pump.vi"("string"="stop", "VISA resource name"=w1080) -> ()  [unwired: 1 out]
                  }
                  frame #3 {
                    n752 = Wait (ms)(milliseconds to wait=u32 500) -> ()  [unwired: 1 out]
                  }
                  frame #4 {
                    n753 = call "Write to pump.vi"("string"="stop", "VISA resource name"=w1084) -> ()  [unwired: 1 out]
                  }
                }
              }
              frame True {
                n754 = flat-sequence {
                  tunnel: w1088 -> [w1098]
                  tunnel: w1089 -> [w1093]
                  tunnel: w1089 -> [w1100]
                  tunnel: w1088 -> [w1101]
                  tunnel: [w1101] -> w1086
                  tunnel: [w1103] -> w1087
                  tunnel: w1086 -> [w1103]
                  tunnel: w1087 -> [w1105]
                  frame #0 {
                    n755 = local read "All Pump Parameters"() -> (w1092:T5)
                    n756 = Unbundle By Name(w1092) -> ("Pump 1"=w1099:T30)
                    n757 = call "Set pump parameters.vi"("Pump write delay (ms)"=w1093, "Volume (uL)"="Ch 1 Inject Volume (uL)", "Rate (uL/h)"="Ch 1 Inject Rate (ul/h)", "Units"=4.0, "Pump #"=1.0, "Pump Parameters In"=w1099, "VISA resource name"=w1098) -> ("Pump Parameters Out"=w1091:T30)  [unwired: 3 in]
                    n758 = Bundle By Name(cluster=w1092, "Pump 1"=w1091) -> (w1090:T5)
                    n759 = local write "All Pump Parameters"(w1090) -> ()
                  }
                  frame #1 {
                    n760 = Wait (ms)(milliseconds to wait=w1100) -> ()  [unwired: 1 out]
                  }
                  frame #2 {
                    n761 = call "Write to pump.vi"("string"="start", "VISA resource name"=w1101) -> ()  [unwired: 1 out]
                  }
                  frame #3 {
                    n762 = Wait (ms)(milliseconds to wait=u32 500) -> ()  [unwired: 1 out]
                  }
                  frame #4 {
                    n763 = call "Write to pump.vi"("string"="start", "VISA resource name"=w1105) -> ()  [unwired: 1 out]
                  }
                }
              }
            }
          }
          frame True {
            n764 = case shown="False" w1107 {
              tunnel: w1108 -> [w1109 w1119]
              frame False {
                n765 = flat-sequence {
                  tunnel: w1109 -> [w1111]
                  frame #0 {
                    n766 = local write "Flushing P1"(FALSE ("Flushing P1")) -> ()
                    n767 = Concatenate Strings("stop" ("string"), "\r") -> (w1113:string)
                    n768 = VISA Write(VISA resource name=w1111, write buffer=w1113) -> ()  [unwired: 1 in, 3 out]
                  }
                  frame #1 {
                    n769 = property on="Clear Volume P1" class="Bool (strict)"("Val(Sgnl)"=TRUE ("Value (Signaling)")) -> ()  [unwired: 2 in, 2 out]
                  }
                }
              }
              frame True {
                n770 = local read "Normal Flow Rate (ul/h) P1"() -> (w1117:dbl)
                n771 = Number To Decimal String(number=w1117) -> (decimal integer string=w1123:string)  [unwired: 1 in]
                n772 = Concatenate Strings("irate  " ("string"), w1123, " u/h" ("string"), "\r") -> (w1121:string)
                n773 = VISA Write(VISA resource name=w1119, write buffer=w1121) -> (VISA resource name out=w1118:refnum<visa-resource-name>)  [unwired: 1 in, 2 out]
                n774 = Concatenate Strings("irun" ("string"), "\r") -> (w1125:string)
                n775 = VISA Write(VISA resource name=w1118, write buffer=w1125) -> ()  [unwired: 1 in, 3 out]
              }
            }
          }
        }
      }
      event "Inject Pump 3": Value Change {
        n776 = event-data() -> ()  [unwired: 7 out]
        n777 = local read "Use Harvard pumps\nfor beads (else Chemyx)"() -> (w1128:bool)
        n778 = case shown="True" w1128 {
          tunnel: "Inject Pump 3" -> [w1132 w1171]
          tunnel: w1127 -> [_ w1170]
          frame False {
            n779 = local read "Pump write delay (ms)"() -> (w1131:dbl)
            n780 = case shown="True" w1132 {
              tunnel: w1131 -> [w1138 w1152]
              tunnel: "Chemyx Syringe Pump Serial Port" -> [w1135 w1151]
              frame False {
                n781 = flat-sequence {
                  tunnel: w1135 -> [w1139]
                  tunnel: [w1139] -> w1136
                  tunnel: w1138 -> [_]
                  tunnel: [w1142] -> w1137
                  tunnel: w1136 -> [w1142]
                  tunnel: w1137 -> [w1143]
                  tunnel: [w1143] -> w1133
                  tunnel: [w1145] -> w1134
                  tunnel: w1133 -> [w1145]
                  tunnel: w1134 -> [w1147]
                  frame #0 {
                    n782 = call "Write to pump.vi"("string"="enter pump3", "VISA resource name"=w1139) -> ()  [unwired: 1 out]
                  }
                  frame #1 {
                    n783 = local read "Pump pause delay (ms)"() -> (w1141:u32)
                    n784 = Wait (ms)(milliseconds to wait=w1141) -> ()  [unwired: 1 out]
                  }
                  frame #2 {
                    n785 = call "Write to pump.vi"("string"="stop", "VISA resource name"=w1143) -> ()  [unwired: 1 out]
                  }
                  frame #3 {
                    n786 = Wait (ms)(milliseconds to wait=u32 0) -> ()  [unwired: 1 out]
                  }
                  frame #4 {
                    n787 = call "Write to pump.vi"("string"="stop", "VISA resource name"=w1147) -> ()  [unwired: 1 out]
                  }
                }
              }
              frame True {
                n788 = flat-sequence {
                  tunnel: w1151 -> [w1161]
                  tunnel: w1152 -> [w1156]
                  tunnel: w1152 -> [w1163]
                  tunnel: w1151 -> [w1164]
                  tunnel: [w1164] -> w1150
                  tunnel: [w1167] -> w1149
                  tunnel: w1150 -> [w1167]
                  tunnel: w1149 -> [w1168]
                  frame #0 {
                    n789 = local read "All Pump Parameters"() -> (w1155:T5)
                    n790 = Unbundle By Name(w1155) -> ("Pump 3"=w1162:T30)
                    n791 = call "Set pump parameters.vi"("Pump write delay (ms)"=w1156, "Volume (uL)"="Ch 3 Inject Volume (uL)", "Rate (uL/h)"="Ch 3 Inject Rate (ul/h)", "Units"=4.0, "Pump #"=3.0, "Pump Parameters In"=w1162, "VISA resource name"=w1161) -> ("Pump Parameters Out"=w1154:T30)  [unwired: 3 in]
                    n792 = Bundle By Name(cluster=w1155, "Pump 3"=w1154) -> (w1153:T5)
                    n793 = local write "All Pump Parameters"(w1153) -> ()
                  }
                  frame #1 {
                    n794 = Wait (ms)(milliseconds to wait=w1163) -> ()  [unwired: 1 out]
                  }
                  frame #2 {
                    n795 = call "Write to pump.vi"("string"="start", "VISA resource name"=w1164) -> ()  [unwired: 1 out]
                  }
                  frame #3 {
                    n796 = Wait (ms)(milliseconds to wait=u32 500) -> ()  [unwired: 1 out]
                  }
                  frame #4 {
                    n797 = call "Write to pump.vi"("string"="start", "VISA resource name"=w1168) -> ()  [unwired: 1 out]
                  }
                }
              }
            }
          }
          frame True {
            n798 = case shown="False" w1171 {
              tunnel: w1170 -> [w1172 w1179]
              frame False {
                n799 = flat-sequence {
                  tunnel: w1172 -> [w1174]
                  frame #0 {
                    n800 = local write "Flushing P3"(FALSE ("Flushing P3")) -> ()
                    n801 = Concatenate Strings("stop" ("string"), "\r") -> (w1176:string)
                    n802 = VISA Write(VISA resource name=w1174, write buffer=w1176) -> ()  [unwired: 1 in, 3 out]
                  }
                  frame #1 {
                    n803 = property on="Clear Volume P3" class="Bool (strict)"("Val(Sgnl)"=TRUE ("Value (Signaling)")) -> ()  [unwired: 2 in, 2 out]
                  }
                }
              }
              frame True {
                n804 = local read "Normal Flow Rate (ul/h) P3"() -> (w1180:dbl)
                n805 = Number To Decimal String(number=w1180) -> (decimal integer string=w1186:string)  [unwired: 1 in]
                n806 = Concatenate Strings("irate  " ("string"), w1186, " u/h" ("string"), "\r") -> (w1184:string)
                n807 = VISA Write(VISA resource name=w1179, write buffer=w1184) -> (VISA resource name out=w1182:refnum<visa-resource-name>)  [unwired: 1 in, 2 out]
                n808 = Concatenate Strings("irun" ("string"), "\r") -> (w1188:string)
                n809 = VISA Write(VISA resource name=w1182, write buffer=w1188) -> ()  [unwired: 1 in, 3 out]
              }
            }
          }
        }
      }
      event "Inject Pump 2": Value Change {
        n810 = event-data() -> ()  [unwired: 7 out]
        n811 = local read "Pump write delay (ms)"() -> (w1192:dbl)
        n812 = flat-sequence {
          tunnel: w1190 -> [w1205]
          tunnel: w1192 -> [w1201]
          tunnel: "Inject Pump 2" -> [_]
          tunnel: w1192 -> [w1207]
          tunnel: w1190 -> [w1208]
          frame #0 {
            n813 = local read "All Pump Parameters"() -> (w1200:T5)
            n814 = Multiply(x=60.0, y="Flush Center Ch Rate (ul/m)") -> (x*y=w1197:dbl)
            n815 = Unbundle By Name(w1200) -> ("Pump 2"=w1206:T30)
            n816 = call "Set pump parameters.vi"("Pump write delay (ms)"=w1201, "Volume (uL)"="Flush Center Ch Volume (uL)", "Rate (uL/h)"=w1197, "Units"=3.0, "Pump #"=2.0, "Pump Parameters In"=w1206, "VISA resource name"=w1205) -> ("Pump Parameters Out"=w1199:T30)  [unwired: 3 in]
            n817 = Bundle By Name(cluster=w1200, "Pump 2"=w1199) -> (w1198:T5)
            n818 = local write "All Pump Parameters"(w1198) -> ()
            n819 = Add(x="Flush Center Ch Volume (uL)", y="Total Volume\nFlushed (uL)") -> (x+y=w1194:dbl)
            n820 = local write "Total Volume\nFlushed (uL)"(w1194) -> ()
          }
          frame #1 {
            n821 = Wait (ms)(milliseconds to wait=w1207) -> ()  [unwired: 1 out]
          }
          frame #2 {
            n822 = call "Write to pump.vi"("string"="start", "VISA resource name"=w1208) -> ()  [unwired: 1 out]
          }
        }
        n823 = local read "Chemyx Syringe Pump Serial Port"() -> (w1190:refnum<visa-resource-name>)
      }
      event "Sample Channel\nFlow": Value Change {
        n824 = event-data() -> ()  [unwired: 7 out]
        n825 = Select(t="irun" ("string"), s="Sample Channel\nFlow", f="stop" ("string")) -> (s? t:f=w1212:string)
        n826 = Concatenate Strings(w1212, "\r") -> (w1215:string)
        n827 = VISA Write(VISA resource name=w1210, write buffer=w1215) -> ()  [unwired: 1 in, 3 out]
      }
      event "Start Flow": Value Change {
        n828 = event-data() -> ()  [unwired: 7 out]
        n829 = local write "Sample Channel\nFlow"(TRUE ("Sample Channel\nFlow")) -> ()
        n830 = local write "Start Flow"(FALSE ("Start Flow")) -> ()
        n831 = Concatenate Strings("irun" ("string"), "\r") -> (w1221:string)
        n832 = VISA Write(VISA resource name=w1217, write buffer=w1221) -> ()  [unwired: 1 in, 3 out]
      }
      event "Stop Flow": Value Change {
        w1223 = FALSE ("Stop Flow")
        n833 = event-data() -> ()  [unwired: 7 out]
        n834 = local write "Stop Flow"(w1223) -> ()
        n835 = local write "Sample Channel\nFlow"(w1223) -> ()
        n836 = Concatenate Strings("stop" ("string"), "\r") -> (w1226:string)
        n837 = VISA Write(VISA resource name=w1224, write buffer=w1226) -> ()  [unwired: 1 in, 3 out]
      }
      event "Flow rate (uL/h)": Value Change {
        n838 = event-data() -> ()  [unwired: 7 out]
        n839 = Number To Decimal String(number="Flow rate (uL/h)") -> (decimal integer string=w1233:string)  [unwired: 1 in]
        n840 = Concatenate Strings("irate  " ("string"), w1233, " u/h" ("string"), "\r") -> (w1232:string)
        n841 = VISA Write(VISA resource name=w1229, write buffer=w1232) -> ()  [unwired: 1 in, 3 out]
      }
      event "Flush Sample": Value Change {
        n842 = event-data() -> ()  [unwired: 7 out]
        n843 = flat-sequence {
          tunnel: w1238 -> [w1266]
          tunnel: [w1246] -> w1237
          tunnel: [w1240] -> w1235
          tunnel: w1237 -> [w1270]
          tunnel: [w1270] -> w1236
          tunnel: w1235 -> [w1269]
          tunnel: w1236 -> [w1275]
          frame #0 {
            # "set paramaters (rate, volume) for flush, clear volume"
            n844 = Number To Decimal String(number="Flush rate (uL/m)") -> (decimal integer string=w1262:string)  [unwired: 1 in]
            n845 = Concatenate Strings("irate  " ("string"), w1262, " u/m" ("string"), "\r") -> (w1264:string)
            n846 = VISA Write(VISA resource name=w1266, write buffer=w1264) -> (VISA resource name out=w1260:refnum<visa-resource-name>)  [unwired: 1 in, 2 out]
            n847 = Reciprocal(x="Flush rate (uL/m)") -> (1/x=w1243:dbl)
            n848 = Number To Decimal String(number="Volume (uL)") -> (decimal integer string=w1251:string)  [unwired: 1 in]
            n849 = Multiply(x="Volume (uL)", y=w1243) -> (x*y=w1242:dbl)
            n850 = Concatenate Strings("tvolume  " ("string"), w1251, " u" ("string"), "\r") -> (w1249:string)
            n851 = Multiply(x=w1242, y=60000.0) -> (x*y=w1240:dbl)
            n852 = VISA Write(VISA resource name=w1260, write buffer=w1249) -> (VISA resource name out=w1248:refnum<visa-resource-name>)  [unwired: 1 in, 2 out]
            n853 = Concatenate Strings("cvolume" ("string"), "\r") -> (w1247:string)
            n854 = VISA Write(VISA resource name=w1248, write buffer=w1247) -> (VISA resource name out=w1258:refnum<visa-resource-name>)  [unwired: 1 in, 2 out]
            n855 = Concatenate Strings("irun" ("string"), "\r") -> (w1256:string)
            n856 = VISA Write(VISA resource name=w1258, write buffer=w1256) -> (VISA resource name out=w1246:refnum<visa-resource-name>)  [unwired: 1 in, 2 out]
          }
          frame #1 {
            # "Have to wait until\nflow is done to reset\nrate"
            n857 = Add(x=w1269, y=100.0) -> (x+y=w1268:dbl)
            n858 = Wait (ms)(milliseconds to wait=w1268) -> ()  [unwired: 1 out]
          }
          frame #2 {
            # "reset flow rate to usual flow rate"
            n859 = local read "Flow rate (uL/h)"() -> (w1281:dbl)
            n860 = Number To Decimal String(number=w1281) -> (decimal integer string=w1279:string)  [unwired: 1 in]
            n861 = Concatenate Strings("irate  " ("string"), w1279, " u/h" ("string"), "\r") -> (w1277:string)
            n862 = VISA Write(VISA resource name=w1275, write buffer=w1277) -> (VISA resource name out=w1271:refnum<visa-resource-name>)  [unwired: 1 in, 2 out]
            n863 = Concatenate Strings("cvolume" ("string"), "\r") -> (w1272:string)
            n864 = VISA Write(VISA resource name=w1271, write buffer=w1272) -> ()  [unwired: 1 in, 3 out]
          }
        }
      }
      event "Flush Pump 3": Value Change {
        n865 = event-data() -> ()  [unwired: 7 out]